vi "UHR-Fleezers Control (host) - Avogadro v1.vi"() -> ()   [LabVIEW 2014] (continued)
                                n2586 = case shown="False" w3926 {
                                tunnel: w3927 -> [_ w3955]
                                tunnel: w3925 -> [w3928 _]
                                frame False {
                                n2587 = flat-sequence {
                                tunnel: w3928 -> [w3929]
                                frame #0 {
                                n2588 = property on="Trap Pos FB SP" class="DigNum (strict)"("Val(Sgnl)"=w3929) -> ()  [unwired: 2 in, 2 out]
                                }
                                frame #1 {
                                n2589 = Wait (ms)(milliseconds to wait=u32 700) -> ()  [unwired: 1 out]
                                }
                                frame #2 {
                                n2590 = local read "Action (%)"() -> (w3934:dbl)
                                n2591 = Absolute Value(x=w3934) -> (abs(x)=w3933:dbl)
                                n2592 = Greater?(x=w3933, y=70.0) -> (0:w3931:bool)
                                n2593 = property on="Remove Action Offset" class="Bool (strict)"("Val(Sgnl)"=w3931) -> ()  [unwired: 2 in, 2 out]
                                }
                                frame #3 {
                                n2594 = for {
                                N: 4 -> [_]
                                n2595 = flat-sequence {
                                frame #0 {
                                n2596 = Wait (ms)(milliseconds to wait=u32 500) -> ()  [unwired: 1 out]
                                }
                                frame #1 {
                                n2597 = local read "Action (%)"() -> (w3940:dbl)
                                n2598 = Absolute Value(x=w3940) -> (abs(x)=w3939:dbl)
                                n2599 = Greater?(x=w3939, y=70.0) -> (0:w3937:bool)
                                n2600 = property on="Remove Action Offset" class="Bool (strict)"("Val(Sgnl)"=w3937) -> ()  [unwired: 2 in, 2 out]
                                }
                                }
                                }
                                }
                                frame #4 {
                                n2601 = Wait (ms)(milliseconds to wait=u32 500) -> ()  [unwired: 1 out]
                                }
                                frame #5 {
                                n2602 = local read "Shift confocal"() -> (w3945:bool)
                                n2603 = local read "Mean"() -> (w3948:dbl)
                                n2604 = Greater?(x=w3948, y=11.0) -> (0:w3944:bool)
                                n2605 = Not(x=w3944) -> (.not. x?=w3943:bool)
                                n2606 = And(x=w3944, y=w3945) -> (x .and. y?=w3946:bool)
                                n2607 = And(x=w3943, y=w3945) -> (x .and. y?=w3942:bool)
                                n2608 = case shown="True" w3946 {
                                frame False {
                                }
                                frame True {
                                n2609 = local read "Confocal X 2 (V)"() -> (w3951:dbl)
                                n2610 = local read "Confocal Y 2 (V)"() -> (w3952:dbl)
                                n2611 = property on="AO2" class="Slide (strict)"("Val(Sgnl)"=w3951) -> ()  [unwired: 2 in, 2 out]
                                n2612 = property on="AO1" class="Slide (strict)"("Val(Sgnl)"=w3952) -> ()  [unwired: 2 in, 2 out]
                                }
                                }
                                n2613 = case shown="True" w3942 {
                                frame False {
                                }
                                frame True {
                                n2614 = local read "Confocal Y 1 (V)"() -> (w3950:dbl)
                                n2615 = local read "Confocal X 1 (V)"() -> (w3949:dbl)
                                n2616 = property on="AO1" class="Slide (strict)"("Val(Sgnl)"=w3950) -> ()  [unwired: 2 in, 2 out]
                                n2617 = property on="AO2" class="Slide (strict)"("Val(Sgnl)"=w3949) -> ()  [unwired: 2 in, 2 out]
                                }
                                }
                                }
                                frame #6 {
                                n2618 = Wait (ms)(milliseconds to wait=u32 1500) -> ()  [unwired: 1 out]
                                }
                                frame #7 {
                                n2619 = property on="Rem fb disp offset" class="Bool (strict)"("Val(Sgnl)"=TRUE ("Value (Signaling)")) -> ()  [unwired: 2 in, 2 out]
                                }
                                }
                                }
                                frame True {
                                n2620 = flat-sequence {
                                tunnel: w3955 -> [w3956]
                                frame #0 {
                                n2621 = property on="Trap Delta (MHz)" class="DigNum (strict)"("Val(Sgnl)"=w3956) -> ()  [unwired: 2 in, 2 out]
                                }
                                frame #1 {
                                n2622 = Wait (ms)(milliseconds to wait=u32 500) -> ()  [unwired: 1 out]
                                }
                                frame #2 {
                                n2623 = local read "Shift confocal"() -> (w3962:bool)
                                n2624 = local read "Mean"() -> (w3963:dbl)
                                n2625 = Greater?(x=w3963, y=11.0) -> (0:w3961:bool)
                                n2626 = And(x=w3961, y=w3962) -> (x .and. y?=w3959:bool)
                                n2627 = Not(x=w3961) -> (.not. x?=w3960:bool)
                                n2628 = And(x=w3960, y=w3962) -> (x .and. y?=w3958:bool)
                                n2629 = case shown="True" w3959 {
                                frame False {
                                }
                                frame True {
                                n2630 = local read "Confocal Y 2 (V)"() -> (w3968:dbl)
                                n2631 = local read "Confocal X 2 (V)"() -> (w3967:dbl)
                                n2632 = property on="AO1" class="Slide (strict)"("Val(Sgnl)"=w3968) -> ()  [unwired: 2 in, 2 out]
                                n2633 = property on="AO2" class="Slide (strict)"("Val(Sgnl)"=w3967) -> ()  [unwired: 2 in, 2 out]
                                }
                                }
                                n2634 = case shown="True" w3958 {
                                frame False {
                                }
                                frame True {
                                n2635 = local read "Confocal Y 1 (V)"() -> (w3966:dbl)
                                n2636 = local read "Confocal X 1 (V)"() -> (w3965:dbl)
                                n2637 = property on="AO2" class="Slide (strict)"("Val(Sgnl)"=w3965) -> ()  [unwired: 2 in, 2 out]
                                n2638 = property on="AO1" class="Slide (strict)"("Val(Sgnl)"=w3966) -> ()  [unwired: 2 in, 2 out]
                                }
                                }
                                }
                                }
                                }
                                }
                                }
                                }
                                }
                                }
                                n2639 = local read "Time (s)"() -> (w3903:dbl)
                                n2640 = Subtract(x=w3904, y=w3903) -> (x-y=w3915:dbl)
                                n2641 = Number To Decimal String(number=w3915, width (-)=i16 0) -> (decimal integer string=w3913:string)
                                n2642 = Concatenate Strings(w3913, " s fluorescence event") -> (w3910:string)
                                n2643 = local read "Messages"() -> (w3911:string)
                                n2644 = local write "Duration (s)"(w3915) -> ()
                                n2645 = call "Update messages.vi"("Message to add"=w3910, "Old message string"=w3911) -> ("New message string"=w3909:string)
                                n2646 = local write "Messages"(w3909) -> ()
                                n2647 = call <vilib>:"Beep.vi"() -> ()  [unwired: 12 in]
                                n2648 = local write "Reset Force"(FALSE ("Force Reset")) -> ()
                                n2649 = local write "Fl. High"(TRUE ("Fl. High")) -> ()
                                n2650 = local write "Waiting"(TRUE ("Waiting")) -> ()
                                }
                                }
                                n2651 = node-c288() -> ()  [unwired: 1 in, 1 out]
                                }
                                n2652 = node-c288(w3882) -> ()  [unwired: 1 out]
                                }
                              }
                            }
                          }
                          n2653 = local read "Trap Delta (MHz)"() -> (w3794:dbl)
                          n2654 = local read "Trap Pos FB SP"() -> (w3792:fxp<+/-,16,1>)
                        }
                      }
                    }
                    frame True {
                      n2655 = flat-sequence {
                        tunnel: w3979 -> [w3989]
                        tunnel: [w3989] -> w3983
                        tunnel: w3982 -> [w3988]
                        tunnel: [w3988] -> w3981
                        tunnel: [w3987] -> w3980
                        tunnel: w3978 -> [w3986]
                        tunnel: [w3985] -> w3977
                        tunnel: w3974 -> [w3984]
                        tunnel: [w3984] -> w3973
                        tunnel: w3983 -> [w4059]
                        tunnel: w3981 -> [w4058]
                        tunnel: w3980 -> [w4057]
                        tunnel: w3977 -> [w4056]
                        tunnel: w3973 -> [w4055]
                        tunnel: [w4056] -> w3976
                        frame #0 {
                          n2656 = call <vilib>:"Beep.vi"() -> ()  [unwired: 3 in, 9 out]
                          n2657 = local write "Waiting"(FALSE ("Waiting")) -> ()
                          n2658 = Increment(x=w3986) -> (x+1=w3985:u8)
                          n2659 = case shown="\"Image\"" w3988 {
                            tunnel: w3985 -> [_ _ w3995]
                            frame "Image" {
                              n2660 = property on="Confocal Image" class="Bool (strict)"("Val(Sgnl)"=TRUE ("Value (Signaling)")) -> ()  [unwired: 2 in, 2 out]
                            }
                            frame "Alarm", Default {
                            }
                            frame "Yank" {
                              n2661 = flat-sequence {
                                tunnel: w3995 -> [w3998]
                                tunnel: [w3997] -> w3994
                                tunnel: ["N Array El"] -> w3993
                                tunnel: w3994 -> [w4012]
                                tunnel: w3993 -> [w4008]
                                frame #0 {
                                n2662 = Multiply(x="Yank Delay (s)", y=1000.0) -> (x*y=w4001:dbl)
                                n2663 = Quotient & Remainder(x=w3998, y="N Array El") -> (x-y*floor(x/y)=w3997:u8)  [unwired: 1 out]
                                n2664 = Wait (ms)(milliseconds to wait=w4001) -> ()  [unwired: 1 out]
                                }
                                frame #1 {
                                n2665 = Random Number (0-1)() -> (number: 0 to 1=w4009:dbl)
                                n2666 = Multiply(x=w4008, y=w4009) -> (x*y=w4007:dbl)
                                n2667 = Round Toward -Infinity(1:w4007) -> (0:w4006:dbl)
                                n2668 = Select(t=w4006, s="Random Choice", f=w4012) -> (s? t:f=w4010:dbl)
                                n2669 = Select(t="Yank to Trap Delta (MHz)", s="Yank to which?", f="Yank to SP") -> (s? t:f=w4003:dbl[])
                                n2670 = Index Array(array=w4003, index=w4010) -> (element=w4013:dbl)
                                n2671 = case shown="False" "Yank to which?" {
                                tunnel: w4013 -> [w4014 w4040]
                                frame False {
                                n2672 = flat-sequence {
                                tunnel: w4014 -> [w4015]
                                frame #0 {
                                n2673 = property on="Trap Pos FB SP" class="DigNum (strict)"("Val(Sgnl)"=w4015) -> ()  [unwired: 2 in, 2 out]
                                }
                                frame #1 {
                                n2674 = Wait (ms)(milliseconds to wait=u32 700) -> ()  [unwired: 1 out]
                                }
                                frame #2 {
                                n2675 = local read "Action (%)"() -> (w4020:dbl)
                                n2676 = Absolute Value(x=w4020) -> (abs(x)=w4019:dbl)
                                n2677 = Greater?(x=w4019, y=70.0) -> (0:w4017:bool)
                                n2678 = property on="Remove Action Offset" class="Bool (strict)"("Val(Sgnl)"=w4017) -> ()  [unwired: 2 in, 2 out]
                                }
                                frame #3 {
                                n2679 = for {
                                N: 4 -> [_]
                                n2680 = flat-sequence {
                                frame #0 {
                                n2681 = Wait (ms)(milliseconds to wait=u32 500) -> ()  [unwired: 1 out]
                                }
                                frame #1 {
                                n2682 = local read "Action (%)"() -> (w4026:dbl)
                                n2683 = Absolute Value(x=w4026) -> (abs(x)=w4025:dbl)
                                n2684 = Greater?(x=w4025, y=70.0) -> (0:w4023:bool)
                                n2685 = property on="Remove Action Offset" class="Bool (strict)"("Val(Sgnl)"=w4023) -> ()  [unwired: 2 in, 2 out]
                                }
                                }
                                }
                                }
                                frame #4 {
                                n2686 = local read "Shift confocal"() -> (w4030:bool)
                                n2687 = local read "Mean"() -> (w4033:dbl)
                                n2688 = Greater?(x=w4033, y=11.0) -> (0:w4029:bool)
                                n2689 = Not(x=w4029) -> (.not. x?=w4028:bool)
                                n2690 = And(x=w4028, y=w4030) -> (x .and. y?=w4027:bool)
                                n2691 = And(x=w4029, y=w4030) -> (x .and. y?=w4031:bool)
                                n2692 = case shown="True" w4031 {
                                frame False {
                                }
                                frame True {
                                n2693 = local read "Confocal X 2 (V)"() -> (w4036:dbl)
                                n2694 = local read "Confocal Y 2 (V)"() -> (w4037:dbl)
                                n2695 = property on="AO2" class="Slide (strict)"("Val(Sgnl)"=w4036) -> ()  [unwired: 2 in, 2 out]
                                n2696 = property on="AO1" class="Slide (strict)"("Val(Sgnl)"=w4037) -> ()  [unwired: 2 in, 2 out]
                                }
                                }
                                n2697 = case shown="True" w4027 {
                                frame False {
                                }
                                frame True {
                                n2698 = local read "Confocal X 1 (V)"() -> (w4034:dbl)
                                n2699 = local read "Confocal Y 1 (V)"() -> (w4035:dbl)
                                n2700 = property on="AO1" class="Slide (strict)"("Val(Sgnl)"=w4035) -> ()  [unwired: 2 in, 2 out]
                                n2701 = property on="AO2" class="Slide (strict)"("Val(Sgnl)"=w4034) -> ()  [unwired: 2 in, 2 out]
                                }
                                }
                                }
                                frame #5 {
                                n2702 = Wait (ms)(milliseconds to wait=u32 1500) -> ()  [unwired: 1 out]
                                }
                                frame #6 {
                                n2703 = property on="Rem fb disp offset" class="Bool (strict)"("Val(Sgnl)"=TRUE ("Value (Signaling)")) -> ()  [unwired: 2 in, 2 out]
                                }
                                }
                                }
                                frame True {
                                n2704 = flat-sequence {
                                tunnel: w4040 -> [w4041]
                                frame #0 {
                                n2705 = property on="Trap Delta (MHz)" class="DigNum (strict)"("Val(Sgnl)"=w4041) -> ()  [unwired: 2 in, 2 out]
                                }
                                frame #1 {
                                n2706 = Wait (ms)(milliseconds to wait=u32 500) -> ()  [unwired: 1 out]
                                }
                                frame #2 {
                                n2707 = local read "Shift confocal"() -> (w4045:bool)
                                n2708 = local read "Mean"() -> (w4043:dbl)
                                n2709 = Greater?(x=w4043, y=11.0) -> (0:w4046:bool)
                                n2710 = Not(x=w4046) -> (.not. x?=w4047:bool)
                                n2711 = And(x=w4047, y=w4045) -> (x .and. y?=w4049:bool)
                                n2712 = And(x=w4046, y=w4045) -> (x .and. y?=w4048:bool)
                                n2713 = case shown="True" w4048 {
                                frame False {
                                }
                                frame True {
                                n2714 = local read "Confocal Y 2 (V)"() -> (w4053:dbl)
                                n2715 = local read "Confocal X 2 (V)"() -> (w4052:dbl)
                                n2716 = property on="AO1" class="Slide (strict)"("Val(Sgnl)"=w4053) -> ()  [unwired: 2 in, 2 out]
                                n2717 = property on="AO2" class="Slide (strict)"("Val(Sgnl)"=w4052) -> ()  [unwired: 2 in, 2 out]
                                }
                                }
                                n2718 = case shown="True" w4049 {
                                frame False {
                                }
                                frame True {
                                n2719 = local read "Confocal X 1 (V)"() -> (w4050:dbl)
                                n2720 = local read "Confocal Y 1 (V)"() -> (w4051:dbl)
                                n2721 = property on="AO2" class="Slide (strict)"("Val(Sgnl)"=w4050) -> ()  [unwired: 2 in, 2 out]
                                n2722 = property on="AO1" class="Slide (strict)"("Val(Sgnl)"=w4051) -> ()  [unwired: 2 in, 2 out]
                                }
                                }
                                }
                                }
                                }
                                }
                                }
                              }
                            }
                          }
                          n2723 = local read "Time (s)"() -> (w3987:dbl)
                          "Fl. High" <- TRUE ("Yanking")
                        }
                        frame #1 {
                          n2724 = local read "Auto F Reset"() -> (w4054:bool)
                          n2725 = case shown="True" w4054 {
                            tunnel: w4059 -> [_ w4063]
                            tunnel: w4058 -> [_ w4062]
                            tunnel: w4057 -> [_ w4061]
                            tunnel: w4055 -> [_ w4060]
                            frame False {
                            }
                            frame True {
                              n2726 = node-c288() -> (w4065:T35)  [unwired: 4 out]
                              n2727 = timed-loop {
                                timing: w4065 -> [_]
                                timing-out: [_] -> w4064
                                tunnel: w4063 -> [w4083]
                                tunnel: w4062 -> [w4082]
                                tunnel: w4061 -> [w4081]
                                tunnel: w4060 -> [w4080]
                                stop <- w4066 stop-if-true
                                n2728 = node-c288() -> ()  [unwired: 2 out]
                                n2729 = local read "Fl. Delta Thresh. (kHz)"() -> (w4074:dbl)
                                n2730 = local read "Fl. Triggered..."() -> (w4079:bool)
                                n2731 = local read "Delta Fl. 1"() -> (w4070:dbl)
                                n2732 = local read "Delta Fl. 2"() -> (w4068:dbl)
                                n2733 = local read "Stop All"() -> (w4077:bool)
                                n2734 = local read "APD to Watch"() -> (w4069:bool)
                                n2735 = Select(t=w4070, s=w4069, f=w4068) -> (s? t:f=w4067:dbl)
                                n2736 = Not(x=w4079) -> (.not. x?=w4078:bool)
                                n2737 = Multiply(x=w4074, y=1000.0) -> (x*y=w4073:dbl)
                                n2738 = Negate(x=w4073) -> (-x=w4072:dbl)
                                n2739 = Less?(x=w4067, y=w4072) -> (x < y?=w4076:bool)
                                n2740 = Compound Arithmetic op=OR(w4076, w4077, w4078, "Reset Force") -> (w4066:bool)
                                n2741 = case shown="True" w4066 {
                                tunnel: w4083 -> [_ w4098]
                                tunnel: w4082 -> [_ w4097]
                                tunnel: w4081 -> [_ w4087]
                                tunnel: w4080 -> [_ w4089]
                                frame False {
                                }
                                frame True {
                                n2742 = local read "Time (s)"() -> (w4088:dbl)
                                n2743 = case shown="\"Yank\"" w4097 {
                                tunnel: w4098 -> [_ w4101]
                                tunnel: w4089 -> [_ w4099]
                                frame "Image", Default {
                                }
                                frame "Yank" {
                                n2744 = flat-sequence {
                                tunnel: [w4107] -> w4102
                                tunnel: w4101 -> [w4107]
                                tunnel: [w4103] -> w4100
                                tunnel: w4099 -> [w4103]
                                tunnel: w4102 -> [w4110]
                                tunnel: w4100 -> [w4108]
                                frame #0 {
                                n2745 = local read "Yank Delay (s)"() -> (w4106:dbl)
                                n2746 = Multiply(x=w4106, y=1000.0) -> (x*y=w4104:dbl)
                                n2747 = Wait (ms)(milliseconds to wait=w4104) -> ()  [unwired: 1 out]
                                }
                                frame #1 {
                                n2748 = local read "Yank to which?"() -> (w4109:bool)
                                n2749 = case shown="False" w4109 {
                                tunnel: w4110 -> [_ w4137]
                                tunnel: w4108 -> [w4111 _]
                                frame False {
                                n2750 = flat-sequence {
                                tunnel: w4111 -> [w4112]
                                frame #0 {
                                n2751 = property on="Trap Pos FB SP" class="DigNum (strict)"("Val(Sgnl)"=w4112) -> ()  [unwired: 2 in, 2 out]
                                }
                                frame #1 {
                                n2752 = Wait (ms)(milliseconds to wait=u32 700) -> ()  [unwired: 1 out]
                                }
                                frame #2 {
                                n2753 = local read "Action (%)"() -> (w4117:dbl)
                                n2754 = Absolute Value(x=w4117) -> (abs(x)=w4116:dbl)
                                n2755 = Greater?(x=w4116, y=70.0) -> (0:w4114:bool)
                                n2756 = property on="Remove Action Offset" class="Bool (strict)"("Val(Sgnl)"=w4114) -> ()  [unwired: 2 in, 2 out]
                                }
                                frame #3 {
                                n2757 = for {
                                N: 4 -> [_]
                                n2758 = flat-sequence {
                                frame #0 {
                                n2759 = Wait (ms)(milliseconds to wait=u32 500) -> ()  [unwired: 1 out]
                                }
                                frame #1 {
                                n2760 = local read "Action (%)"() -> (w4123:dbl)
                                n2761 = Absolute Value(x=w4123) -> (abs(x)=w4122:dbl)
                                n2762 = Greater?(x=w4122, y=70.0) -> (0:w4120:bool)
                                n2763 = property on="Remove Action Offset" class="Bool (strict)"("Val(Sgnl)"=w4120) -> ()  [unwired: 2 in, 2 out]
                                }
                                }
                                }
                                }
                                frame #4 {
                                n2764 = local read "Shift confocal"() -> (w4128:bool)
                                n2765 = local read "Mean"() -> (w4130:dbl)
                                n2766 = Greater?(x=w4130, y=11.0) -> (0:w4127:bool)
                                n2767 = Not(x=w4127) -> (.not. x?=w4126:bool)
                                n2768 = And(x=w4127, y=w4128) -> (x .and. y?=w4125:bool)
                                n2769 = And(x=w4126, y=w4128) -> (x .and. y?=w4124:bool)
                                n2770 = case shown="True" w4125 {
                                frame False {
                                }
                                frame True {
                                n2771 = local read "Confocal Y 2 (V)"() -> (w4134:dbl)
                                n2772 = local read "Confocal X 2 (V)"() -> (w4133:dbl)
                                n2773 = property on="AO2" class="Slide (strict)"("Val(Sgnl)"=w4133) -> ()  [unwired: 2 in, 2 out]
                                n2774 = property on="AO1" class="Slide (strict)"("Val(Sgnl)"=w4134) -> ()  [unwired: 2 in, 2 out]
                                }
                                }
                                n2775 = case shown="True" w4124 {
                                frame False {
                                }
                                frame True {
                                n2776 = local read "Confocal X 1 (V)"() -> (w4131:dbl)
                                n2777 = local read "Confocal Y 1 (V)"() -> (w4132:dbl)
                                n2778 = property on="AO1" class="Slide (strict)"("Val(Sgnl)"=w4132) -> ()  [unwired: 2 in, 2 out]
                                n2779 = property on="AO2" class="Slide (strict)"("Val(Sgnl)"=w4131) -> ()  [unwired: 2 in, 2 out]
                                }
                                }
                                }
                                frame #5 {
                                n2780 = Wait (ms)(milliseconds to wait=u32 1500) -> ()  [unwired: 1 out]
                                }
                                frame #6 {
                                n2781 = property on="Rem fb disp offset" class="Bool (strict)"("Val(Sgnl)"=TRUE ("Value (Signaling)")) -> ()  [unwired: 2 in, 2 out]
                                }
                                }
                                }
                                frame True {
                                n2782 = flat-sequence {
                                tunnel: w4137 -> [w4138]
                                frame #0 {
                                n2783 = property on="Trap Delta (MHz)" class="DigNum (strict)"("Val(Sgnl)"=w4138) -> ()  [unwired: 2 in, 2 out]
                                }
                                frame #1 {
                                n2784 = Wait (ms)(milliseconds to wait=u32 500) -> ()  [unwired: 1 out]
                                }
                                frame #2 {
                                n2785 = local read "Shift confocal"() -> (w4144:bool)
                                n2786 = local read "Mean"() -> (w4146:dbl)
                                n2787 = Greater?(x=w4146, y=11.0) -> (0:w4143:bool)
                                n2788 = Not(x=w4143) -> (.not. x?=w4142:bool)
                                n2789 = And(x=w4143, y=w4144) -> (x .and. y?=w4141:bool)
                                n2790 = And(x=w4142, y=w4144) -> (x .and. y?=w4140:bool)
                                n2791 = case shown="True" w4141 {
                                frame False {
                                }
                                frame True {
                                n2792 = local read "Confocal Y 2 (V)"() -> (w4150:dbl)
                                n2793 = local read "Confocal X 2 (V)"() -> (w4149:dbl)
                                n2794 = property on="AO2" class="Slide (strict)"("Val(Sgnl)"=w4149) -> ()  [unwired: 2 in, 2 out]
                                n2795 = property on="AO1" class="Slide (strict)"("Val(Sgnl)"=w4150) -> ()  [unwired: 2 in, 2 out]
                                }
                                }
                                n2796 = case shown="True" w4140 {
                                frame False {
                                }
                                frame True {
                                n2797 = local read "Confocal Y 1 (V)"() -> (w4148:dbl)
                                n2798 = local read "Confocal X 1 (V)"() -> (w4147:dbl)
                                n2799 = property on="AO2" class="Slide (strict)"("Val(Sgnl)"=w4147) -> ()  [unwired: 2 in, 2 out]
                                n2800 = property on="AO1" class="Slide (strict)"("Val(Sgnl)"=w4148) -> ()  [unwired: 2 in, 2 out]
                                }
                                }
                                }
                                }
                                }
                                }
                                }
                                }
                                }
                                }
                                n2801 = local read "Messages"() -> (w4096:string)
                                n2802 = Subtract(x=w4088, y=w4087) -> (x-y=w4094:dbl)
                                "Duration (s)" <- w4094
                                n2803 = Number To Decimal String(number=w4094, width (-)=i16 0) -> (decimal integer string=w4092:string)
                                n2804 = Concatenate Strings(w4092, " s fluorescence event." ("string")) -> (w4090:string)
                                n2805 = call "Update messages.vi"("Message to add"=w4090, "Old message string"=w4096) -> ("New message string"=w4095:string)
                                n2806 = local write "Reset Force"(FALSE ("Reset Force")) -> ()
                                n2807 = local write "Waiting"(TRUE ("Waiting")) -> ()
                                n2808 = local write "Messages"(w4095) -> ()
                                n2809 = local write "Fl. High"(FALSE ("Fl. High")) -> ()
                                n2810 = call <vilib>:"Beep.vi"() -> ()  [unwired: 3 in, 9 out]
                                }
                                }
                                n2811 = node-c288() -> ()  [unwired: 2 out]
                              }
                              n2812 = node-c288(w4064) -> ()  [unwired: 1 out]
                            }
                          }
                        }
                      }
                      n2813 = local read "Trap Delta (MHz)"() -> (w3979:dbl)
                      n2814 = local read "Trap Pos FB SP"() -> (w3974:fxp<+/-,16,1>)
                    }
                  }
                }
                frame #1 {
                  n2815 = local read "Stop All"() -> (w4160:bool)
                  n2816 = local read "Fl. Triggered..."() -> (w4158:bool)
                  n2817 = Not(x=w4158) -> (.not. x?=w4159:bool)
                  n2818 = Or(x=w4159, y=w4160) -> (x .or. y?=w4157:bool)
                }
              }
              n2819 = case shown="True" w3751 {
                frame False {
                }
                frame True {
                  n2820 = local read "Confocal Y 1 (V)"() -> (w3761:dbl)
                  n2821 = local read "Confocal X 1 (V)"() -> (w3760:dbl)
                  n2822 = property on="AO2" class="Slide (strict)"("Val(Sgnl)"=w3760) -> ()  [unwired: 2 in, 2 out]
                  n2823 = property on="AO1" class="Slide (strict)"("Val(Sgnl)"=w3761) -> ()  [unwired: 2 in, 2 out]
                }
              }
              n2824 = case shown="True" w3751 {
                frame False {
                }
                frame True {
                  w3759 = FALSE ("Fl. High")
                  n2825 = local write "Waiting"(w3759) -> ()
                  n2826 = local write "Fl. High"(w3759) -> ()
                }
              }
              n2827 = node-c288() -> ()  [unwired: 2 out]
            }
            n2828 = node-c288(w3749) -> ()  [unwired: 1 out]
          }
        }
      }
      event "Start assembly line": Value Change {
        n2829 = event-data() -> ()  [unwired: 7 out]
        n2830 = case shown="True" "Start assembly line" {
          tunnel: w4166 -> [_ w4167]
          frame False {
          }
          frame True {
            n2831 = flat-sequence {
              tunnel: w4167 -> [w4172]
              tunnel: [w4171] -> w4169
              tunnel: w4169 -> [w4204]
              tunnel: [w4203] -> w4168
              tunnel: w4168 -> [w4206]
              tunnel: w4167 -> [w4225]
              frame #0 {
                w4170 = TRUE ("Value (Signaling)")
                n2832 = property on="Green Laser ON" class="Bool (strict)"("Val(Sgnl)"=w4170) -> ()  [unwired: 2 in, 2 out]
                "AL Running" <- w4170
              }
              frame #1 {
                n2833 = node-c288() -> (w4174:T35)  [unwired: 4 in]
                n2834 = timed-loop {
                  timing: w4174 -> [_]
                  timing-out: [_] -> w4173
                  tunnel: w4172 -> [w4182]
                  tunnel: [w4177] -> w4171
                  stop <- w4178 stop-if-true
                  n2835 = node-c288() -> ()  [unwired: 1 in, 1 out]
                  n2836 = local read "APD rates cluster"() -> (w4176:T1)
                  n2837 = Multiply(x="Cy3 Fl.  Thresh. (kHz)", y=1000.0) -> (x*y=w4185:dbl)
                  n2838 = Unbundle By Name(w4176) -> ("APD 1 Rate (Hz)"=w4175:dbl)
                  n2839 = Greater?(x=w4175, y=w4185) -> (0:w4181:bool)
                  n2840 = case shown="True" w4181 {
                    tunnel: w4182 -> [_ w4188]
                    tunnel: [TRUE ("Stage Moving") w4187] -> w4180
                    frame False {
                    }
                    frame True {
                      n2841 = flat-sequence {
                        tunnel: w4188 -> [w4193]
                        tunnel: [w4198] -> w4187
                        frame #0 {
                          n2842 = Multiply(x="AL Delay (s)", y=u32 1000) -> (x*y=w4190:u32)
                          n2843 = Wait (ms)(milliseconds to wait=w4190) -> ()  [unwired: 1 out]
                        }
                        frame #1 {
                          n2844 = property on="Green Laser ON" class="Bool (strict)"("Val(Sgnl)"=FALSE ("Value (Signaling)")) -> ()  [unwired: 2 in, 2 out]
                        }
                        frame #2 {
                          # "upper spot"
                          n2845 = local read "Saved Stage Positions"() -> (w4196:dbl[][])
                          n2846 = local write "Stage Moving"(TRUE ("Stage Moving")) -> ()
                          n2847 = call "move to saved stage position.vi"("Stage VISA resource name in"=w4193, "Position"=5, "Saved Stage Positions"=w4196) -> ("error out"=w4194:errorcluster)  [unwired: 1 in, 1 out]
                          n2848 = local write "Stage Control Serial Error"(w4194) -> ()
                        }
                        frame #3 {
                          w4198 = FALSE ("Stage Moving")
                          n2849 = call <vilib>:"Beep.vi"() -> ()  [unwired: 3 in, 9 out]
                          n2850 = local write "Stage Moving"(w4198) -> ()
                        }
                      }
                    }
                  }
                  n2851 = local read "Stop assembly line"() -> (w4177:bool)
                  n2852 = Not(x=w4180) -> (.not. x?=w4179:bool)
                  n2853 = node-c288() -> ()  [unwired: 1 in, 1 out]
                  n2854 = Or(x=w4179, y=w4177) -> (x .or. y?=w4178:bool)
                }
                n2855 = node-c288(w4173) -> ()  [unwired: 1 out]
              }
              frame #2 {
                n2856 = Not(x=w4204) -> (.not. x?=w4203:bool)
                n2857 = case shown="True" w4203 {
                  frame False {
                  }
                  frame True {
                    n2858 = property on="Red Laser ON" class="Bool (strict)"("Val(Sgnl)"=TRUE ("Value (Signaling)")) -> ()  [unwired: 2 in, 2 out]
                  }
                }
              }
              frame #3 {
                n2859 = node-c288() -> (w4208:T35)  [unwired: 4 in]
                n2860 = timed-loop {
                  timing: w4208 -> [_]
                  timing-out: [_] -> w4207
                  tunnel: [w4211] -> _
                  tunnel: w4206 -> [w4211]
                  stop <- "Stop assembly line" stop-if-true
                  n2861 = node-c288() -> ()  [unwired: 1 in, 1 out]
                  n2862 = local read "APD rates cluster"() -> (w4210:T1)
                  n2863 = Multiply(x="Cy5 Fl.  Thresh. (kHz)", y=1000.0) -> (x*y=w4217:dbl)
                  n2864 = Unbundle By Name(w4210) -> ("APD 2 Rate (Hz)"=w4209:dbl)
                  n2865 = Greater?(x=w4209, y=w4217) -> (0:w4214:bool)
                  n2866 = And(x=w4214, y=w4211) -> (x .and. y?=w4212:bool)
                  n2867 = case shown="True" w4212 {
                    frame False {
                    }
                    frame True {
                      n2868 = property on="Green Laser ON" class="Bool (strict)"("Val(Sgnl)"=TRUE ("Value (Signaling)")) -> ()  [unwired: 2 in, 2 out]
                    }
                  }
                  n2869 = node-c288() -> ()  [unwired: 1 in, 1 out]
                }
                n2870 = node-c288(w4207) -> ()  [unwired: 1 out]
              }
              frame #4 {
                w4224 = FALSE ("Value (Signaling)")
                # "lower spot"
                n2871 = local read "Saved Stage Positions"() -> (w4228:dbl[][])
                n2872 = property on="Red Laser ON" class="Bool (strict)"("Val(Sgnl)"=w4224) -> ()  [unwired: 2 in, 2 out]
                n2873 = property on="Green Laser ON" class="Bool (strict)"("Val(Sgnl)"=w4224) -> ()  [unwired: 2 in, 2 out]
                n2874 = local write "Stage Moving"(TRUE ("Stage Moving")) -> ()
                n2875 = local write "Stop assembly line"(FALSE ("Stop assembly line")) -> ()
                n2876 = call "move to saved stage position.vi"("Stage VISA resource name in"=w4225, "Position"=3, "Saved Stage Positions"=w4228) -> ("error out"=w4227:errorcluster)  [unwired: 1 in, 1 out]
                n2877 = local write "Stage Control Serial Error"(w4227) -> ()
              }
              frame #5 {
                w4230 = FALSE ("Stage Moving")
                n2878 = local write "Stage Moving"(w4230) -> ()
                n2879 = local write "AL Running"(w4230) -> ()
                n2880 = call <vilib>:"Beep.vi"() -> ()  [unwired: 3 in, 9 out]
              }
            }
          }
        }
      }
      event "Stop All": Value Change {
        n2881 = event-data() -> ()  [unwired: 7 out]
        n2882 = local read "Stop All"() -> (w4231:bool)
      }
    }
    n2883 = node-c288() -> ()  [unwired: 2 out]
  }
  n2884 = node-c288(w64) -> ()  [unwired: 1 out]
  n2885 = node-c288(w66) -> ()  [unwired: 1 out]
  n2886 = node-c288(w55) -> ()  [unwired: 1 out]
  n2887 = property on="Saved trap pos" class="WFGraph (strict)"("Visible"=FALSE) -> ()  [unwired: 2 in, 2 out]
  n2888 = property on="Trap Delta Graph" class="WFGraph (strict)"("Visible"=TRUE) -> ()  [unwired: 2 in, 2 out]
  n2889 = disable-structure shown="Disabled" {
    disable-tunnel: w58 -> [w4233 _]
    disable-tunnel: w57 -> [w4232 _]
    frame Disabled {
      n2890 = VISA Close(VISA resource name=w4233, error in (no error)=w4232) -> (error out=w4234:errorcluster)
      n2891 = call <vilib>:"Simple Error Handler.vi"("error in (no error)"=w4234) -> ()  [unwired: 1 in, 8 out]
    }
    frame Enabled {
    }
  }
  n2892 = disable-structure shown="Disabled" {
    disable-tunnel: [w4242 _] -> w19
    disable-tunnel: [w4238 _] -> w18
    disable-tunnel: [w4237 _] -> w17
    disable-tunnel: [w4236 _] -> w16
    disable-tunnel: [w4235 _] -> w15
    frame Disabled {
      # "n samples needed for data"
      n2893 = Unbundle By Name("sound format") -> ("sample rate (S/s)"=w4238:dbl)
      n2894 = call <vilib>:"Sound Output Configure.vi"("number of samples/ch"="number of samples/ch", "sample mode"="sample mode", "sound format"="sound format", "device ID"="device ID") -> ("task ID"=w4242:T52)  [unwired: 6 in, 1 out]
      n2895 = local read "DMA Update Period (s)"() -> (w4239:dbl)
      n2896 = Multiply(x=w4239, y=w4238) -> (x*y=w4237:dbl)
      n2897 = for "Sound time base" {
        N: w4237 -> [_]
        tunnel: [w4246] -> w4240 mode=indexing
        i -> [w4246]
      }
      n2898 = Reciprocal(x=w4238) -> (1/x=w4236:dbl)
      n2899 = Multiply(x=w4240, y=w4236) -> (x*y=w4235:dbl[])
    }
    frame Enabled {
    }
  }
  n2900 = timed-loop "Main data acquisition loop (get data, process data for display, and save data to disk)" {
    tunnel: w14 -> [w4322]
    tunnel: w27 -> [w4321]
    tunnel: [w4580] -> w78
    tunnel: [w4575] -> w77
    timing: w71 -> [_]
    timing-out: [_] -> w70
    tunnel: w49 -> [w4487]
    tunnel: [w4377] -> w20
    tunnel: w19 -> [w4376]
    tunnel: w18 -> [w4374]
    tunnel: w17 -> [w4373]
    tunnel: w16 -> [w4372]
    tunnel: w15 -> [w4371]
    stop <- "Stop All" stop-if-true
    w4270 = 2.0
    w4296 = 3276.7
    w4434 = "Initialize"
    # "Modified by Ronen 180227: Allows for taking confocal image by moving the piezo trap with a bead inside and using trap 1 (AOM) with very low intensity to measure it"
    # "Cursor control of MCL trap position"
    # "Values for plotting"
    # "Added by Ronen - the limits imposed on amplitudes sent to AOM\nare not explicitly imposed when using intensity feedback. At amplitude of \n~48% FB intensity is ~1.8, if while feedback is on the value passes 1.8, feedback\nis turned off (indication that feedback algorithm overshoots)."
    # "List of channels in order (X or Y only):\nT1 X (mV)\nT2 X (mV)\nT1 X (nm)\nT2 X (nm)\nT1 FX (pN)\nT2 FX (pN)\nPosition Difference (nm)\nAPD1\nAPD2\nAPD3"
    # "T2 sum"
    # "T1 sum"
    n2901 = node-c288() -> ()  [unwired: 2 out]
    n2902 = First Call?() -> (First Call?: T/F=w4447:bool)
    n2903 = Or(x="Reset", y=w4447) -> (x .or. y?=w4448:bool)
    n2904 = Or(x="Start AOD Scan", y="Trap Raster Scan") -> (x .or. y?=w4534:bool)
    n2905 = case "Reset data stream (manual reset or at begining of some rastering and imaging)" shown="True" w4448 {
      tunnel: w4322 -> [w5386 w5394]
      tunnel: w4321 -> [w5385 w5393]
      tunnel: [w5386 w5388] -> w4352
      tunnel: [w5385 w5387] -> w4353
      frame False {
      }
      frame True {
        w5391 = TRUE ("AI to FIFO")
        n2906 = call "reset FPGA DMA.vi"("error in"=w5393, "FPGA VI Reference In"=w5394) -> ("error out"=w5389:errorcluster, "FPGA VI Reference Out"=w5390:T41)
        n2907 = local write "Overflow (data lost)"(FALSE ("Overflow (data lost)")) -> ()
        n2908 = xnode "Read/Write Control"("FPGA VI Reference In"=w5390, "error in"=w5389, "AI to FIFO"=w5391, "APD to FIFO"=w5391) -> ("FPGA VI Reference Out"=w5388:T41, "error out"=w5387:errorcluster)
      }
    }
    n2909 = case "Start active calibration (oscillate traps precisely)" shown="True" "Active Cal" {
      tunnel: w4353 -> [w4681 w4689]
      tunnel: w4352 -> [w4680 w4690]
      tunnel: [w4681 w4686] -> w4351
      tunnel: [w4680 w4687] -> w4350
      frame False {
      }
      frame True {
        w4682 = TRUE ("APD to FIFO")
        n2910 = call "reset FPGA DMA.vi"("error in"=w4689, "FPGA VI Reference In"=w4690) -> ("error out"=w4683:errorcluster, "FPGA VI Reference Out"=w4684:T41)
        n2911 = local write "Active Cal"(FALSE ("Active Cal")) -> ()
        n2912 = local write "Save Calibration"(TRUE ("Save Calibration")) -> ()
        n2913 = xnode "Read/Write Control"("FPGA VI Reference In"=w4684, "error in"=w4683, "AI to FIFO"=w4682, "APD to FIFO"=w4682) -> ("FPGA VI Reference Out"=w4687:T41, "error out"=w4686:errorcluster)
      }
    }
    n2914 = case shown="True" "Read Lateness and Rel Phase" {
      tunnel: w4322 -> [w4905 w4936]
      tunnel: w4321 -> [w4906 w4935]
      tunnel: [w4905 w4907] -> w4292
      tunnel: [w4906 w4908] -> w4523
      frame False {
      }
      frame True {
        n2915 = xnode "Read/Write Control"("FPGA VI Reference In"=w4936, "error in"=w4935) -> ("FPGA VI Reference Out"=w4907:T41, "error out"=w4908:errorcluster, "GI Relative phase"=→"GI relative phase":i16, "Relative phase"=→"Relative phase (AI1)":i16, "AI Late Counter"=→"Late Counter (AI1)":u8, "GI Late Counter"=→"GI Late Counter":u8, "MCL Late Counter"=→"MCL Late Counter":u8, "MCL Relative Phase"=→"Relative Phase (MCL)":i16, "APD Acq Relative Phase"=→"APD Acq Relative Phase":i16, "APD 1 Gate Relative Phase"=→"APD 1 Gate Relative Phase":i16, "APD 2 Gate Relative Phase"=→"APD 2 Gate Relative Phase":i16, "APD Acq Late Counter"=→"APD Acq Late Counter":u8, "APD 1 Gate Late Counter"=→"APD 1 Gate Late Counter":u8, "APD 2 Gate Late Counter"=→"APD 2 Gate Late Counter":u8, "Green FB Relative Phase"=→"Relative phase (Green FB)":i16, "GI Relative phase 2"=→"GI relative phase 2":i16, "GI Late Counter 2"=→"GI Late Counter 2":u8, "Trap Pos FIFO Timeout"=→"Trap Pos FIFO Timeout":u16, "Trap AI FIFO Timeout"=→"Trap AI FIFO Timeout":u16, "RI Late Counter"=→"RI Late Counter":u8, "RI Relative phase"=→"RI relative phase":i16, "Green Late Counter"=→"Green AI Late Counter":u8, "BI Late Counter (AO)"=→"Late Counter (BI AO)":u8, "Blue Late Counter (D)"=→"Late Counter (BI DO)":u8, "BI Relative phase (AO)"=→"Relative phase (BI AO)":i16, "BI Relative phase (D)"=→"Relative phase (BI DO)":i16, "APD 3 Gate Late Counter"=→"APD 3 Gate Late Counter":u8, "APD 3 Gate Relative Phase"=→"APD 3 Gate Relative Phase":i16)
      }
    }
    n2916 = Compound Arithmetic op=OR("Start MCL Scan", "Confocal Image", "Confocal Linescan") -> (w4320:bool)
    n2917 = And(x="Save Data (MCL)", y=w4320) -> (x .and. y?=w4553:bool)
    n2918 = case "Start AOM raster scan" shown="False" w4534 {
      tunnel: w4350 -> [w5245 w5255]
      tunnel: w4351 -> [w5244 w5254]
      tunnel: [w5245 w5248] -> w4556
      tunnel: [w5244 w5247] -> w4555
      frame False {
      }
      frame True {
        n2919 = case shown="True" "Restart DMA? (AOD)" {
          tunnel: [w5284 w5286] -> w5249
          tunnel: [w5283 w5285] -> w5250
          tunnel: w5255 -> [w5284 w5288]
          tunnel: w5254 -> [w5283 w5287]
          frame False {
          }
          frame True {
            n2920 = local write "Overflow (data lost)"(FALSE ("Overflow (data lost)")) -> ()
            n2921 = call "reset FPGA DMA.vi"("error in"=w5287, "FPGA VI Reference In"=w5288) -> ("error out"=w5285:errorcluster, "FPGA VI Reference Out"=w5286:T41)
          }
        }
        n2922 = local write "Trap Raster Scan"(FALSE ("Trap Raster Scan")) -> ()
        n2923 = case shown="True" "Move MCL Also?" {
          tunnel: w5250 -> [w5258 w5278]
          tunnel: w5249 -> [w5259 w5279]
          tunnel: [w5257 w5282] -> w5248
          tunnel: [w5256 w5281] -> w5247
          frame False {
            w5260 = TRUE ("AI to FIFO")
            n2924 = xnode "Read/Write Control"("FPGA VI Reference In"=w5259, "error in"=w5258, "AI to FIFO"=w5260, "APD to FIFO"=w5260, "Start scan"=w5260) -> ("FPGA VI Reference Out"=w5257:T41, "error out"=w5256:errorcluster)
          }
          frame True {
            w5276 = FALSE ("1D or 2D Scan?")
            w5280 = TRUE ("AI to FIFO")
            n2925 = local read "Scan Range (nm)"() -> (w5273:dbl)
            n2926 = local read "Scan steps (AOD)"() -> (w5267:u64)
            n2927 = local read "Total Counts (ticks)"() -> (w5268:u16)
            n2928 = local read "Cycles/step (AOD)"() -> (w5266:u64)
            n2929 = local read "Number of F/B Scans (AOD)"() -> (w5275:u16)
            n2930 = Bundle("Scan Range (nm)"=w5273, "MCL Step Position Ratio"="MCL Step Position Ratio", "MCL/AOM Scale Tweak"="MCL/AOM Scale Tweak", "MCL X Cal (nm/V)"="MCL X Cal (nm/V)", "MCL Step Increment (V_int)"="MCL Step Increment (V_int)", "Total Counts (ticks)"=w5268, "Scan steps (AOD)"=w5267, "Cycles/step (AOD)"=w5266) -> (w5265:T60)  [unwired: 1 in]
            n2931 = call "Calculate MCL scan parameters.vi"("Input parameters"=w5265) -> ("Scan steps(MCL)"=w5264:dbl, "Scan Freq. Increment (MCL)"=w5263:dbl, "MCL Count"=w5262:dbl)
            "MCL Count" <- w5262
            n2932 = xnode "Read/Write Control"("FPGA VI Reference In"=w5279, "error in"=w5278, "Scan steps (MCL)"=w5264, "Number of scans (MCL)"=w5275, "Cycles per step (MCL)"=u64 1, "Scan freq.  increment (MCL)"=w5263, "1D or 2D Scan?"=w5276, "MCL Scan Axis"=w5276, "Cont. Scan (MCL)"=w5276, "MCL count"=w5262) -> ("FPGA VI Reference Out"=w5261:T41, "error out"=w5277:errorcluster)
            n2933 = local write "MCL Scanning"(w5280) -> ()
            n2934 = local write "wait to reset values"(w5280) -> ()
            n2935 = xnode "Read/Write Control"("FPGA VI Reference In"=w5261, "error in"=w5277, "AI to FIFO"=w5280, "APD to FIFO"=w5280, "Start scan"=w5280, "Start scan (MCL)"=w5280) -> ("FPGA VI Reference Out"=w5282:T41, "error out"=w5281:errorcluster)
          }
        }
        "Raster Scanning..." <- TRUE ("Scanning...")
      }
    }
    n2936 = case "Start MCL raster scan" shown="True" w4320 {
      tunnel: w4556 -> [w5123 w5141]
      tunnel: w4555 -> [w5122 w5140]
      tunnel: [w5123 w5136] -> w4486
      tunnel: [w5122 w5135] -> w4485
      tunnel: [FALSE w5134] -> w4539
      tunnel: "Start MCL Scan" -> [_ w5131]
      tunnel: "Confocal Image" -> [_ w5130]
      tunnel: "Confocal Linescan" -> [_ _]
      frame False {
      }
      frame True {
        w5134 = TRUE
        n2937 = case shown="True" "Restart DMA? (MCL)" {
          tunnel: [w5217 w5219] -> w5139
          tunnel: [w5216 w5218] -> w5138
          tunnel: w5141 -> [w5217 w5222]
          tunnel: w5140 -> [w5216 w5221]
          frame False {
          }
          frame True {
            n2938 = call "reset FPGA DMA.vi"("error in"=w5221, "FPGA VI Reference In"=w5222) -> ("error out"=w5218:errorcluster, "FPGA VI Reference Out"=w5219:T41)
            n2939 = local write "Overflow (data lost)"(FALSE ("Overflow (data lost)")) -> ()
          }
        }
        n2940 = case shown="False" w5131 {
          tunnel: w5130 -> [w5144 _]
          frame False {
            n2941 = property on="Confocal Image" class="Bool (strict)"("Value"=FALSE ("Start Confocal Map")) -> ()  [unwired: 2 in, 2 out]
            n2942 = property on="2D or 1D Scan" class="Bool (strict)"("Val(Sgnl)"=w5144) -> ()  [unwired: 2 in, 2 out]